vi "2_VisualizeModulePositioning2_Nolan.vi"(0 "Placement Monitor":T1(plugin-control)=refnum, 1 "Calibrated positions of fiducials [mm]":dbl[][](array[numeric])=[[-658.867386146, 115.937184375, -18.342965965], [-563.38738772, 115.95451918, -18.342965965], [-563.369748267, 18.796520782, -18.342965965], [-658.849746693, 18.779185977, -18.342965965], [-560.867387761, 115.954976697, -18.342965965], [-465.387389335, 115.972311502, -18.342965965], [-465.369749882, 18.814313103, -18.342965965], [-560.849748308, 18.796978298, -18.342965965], [-462.867389377, 115.972769019, -18.342965965], [-367.38739095, 115.990103824, -18.342965965], [-367.369751497, 18.832105425, -18.342965965], [-462.849749923, 18.81477062, -18.342965965], [-364.867390992, 115.990561341, -18.342965965], [-269.387392565, 116.007896146, -18.342965965], [-269.369753112, 18.849897747, -18.342965965], [-364.849751539, 18.832562942, -18.342965965], [-266.867392607, 116.008353663, -18.342965965], [-171.38739418, 116.025688468, -18.342965965], [-171.369754727, 18.867690069, -18.342965965], [-266.849753154, 18.850355264, -18.342965965], [-168.867394222, 116.026145985, -18.342965965], [-73.387395796, 116.04348079, -18.342965965], [-73.369756342, 18.885482391, -18.342965965], [-168.849754769, 18.868147586, -18.342965965], [-70.867395837, 116.043938306, -18.342965965], [24.612602589, 116.061273111, -18.342965965], [24.630242042, 18.903274713, -18.342965965], [-70.849756384, 18.885939908, -18.342965965], [27.132602548, 116.061730628, -18.342965965], [122.612600974, 116.079065433, -18.342965965], [122.630240427, 18.921067035, -18.342965965], [27.150242001, 18.90373223, -18.342965965], [125.132600933, 116.07952295, -18.342965965], [220.612599359, 116.096857755, -18.342965965], [220.630238812, 18.938859356, -18.342965965], [125.150240386, 18.921524551, -18.342965965], [223.132599318, 116.097315272, -18.342965965], [318.612597744, 116.114650077, -18.342965965], [318.630237197, 18.956651678, -18.342965965], [223.150238771, 18.939316873, -18.342965965], [321.132597702, 116.115107594, -18.342965965], [416.612596129, 116.132442399, -18.342965965], [416.630235582, 18.974444, -18.342965965], [321.150237156, 18.957109195, -18.342965965], [419.132596087, 116.132899916, -18.342965965], [514.612594514, 116.150234721, -18.342965965], [514.630233967, 18.992236322, -18.342965965], [419.15023554, 18.974901517, -18.342965965], [517.132594472, 116.150692238, -18.342965965], [612.612592899, 116.168027043, -18.342965965], [612.630232352, 19.010028644, -18.342965965], [517.150233925, 18.992693839, -18.342965965]], 2 "XYZ .NET Refnum in":refnum<k24>, 3 "Axis Speeds":T10={"X [mm/s]"=25.0, "Y [mm/s]"=25.0, "Z [mm/s]"=25.0}, 4 "Module fiducial marker":T7=enum."Mark C", 5 "N modules":i32=13, 6 "Sensor Pattern":T8(ring)=enum."ATLAS12", 7 "error in (no error)":errorcluster, 8 "Templates path":path=path "C:/Users/Aerotech/Documents/BNL_ThermomechanicalStave", 9 "Calibration [um/pix]":dbl=1.55, 10 "Current Build Phase":refnum<vi>, 11 "Temperature":refnum<vi>, 12 "Module #":refnum<vi>, 13 "Placement tolerance [um]":dbl=25.0, 14 "Tape Type":T5=enum."Axial (Sutcliffe NP49-01-100 01-Mar-16)", 16 "Module Report":refnum<vi>, 17 "Base notes":string, 18 "Reports path":path=path "C:/Users/Aerotech/cernbox/BNL/Stave Assembly Records/2017-05-15/ModulePlacement") -> (19 "Recalibrated??":bool, 22 "XYZ .NET Refnum out":refnum<k24>, 27 "error out":errorcluster)   [LabVIEW 2016]
uses:
  Utils/Controls/All_Enums/Enum_TypeDef_FidMarkers.ctl
  C:/Users/Aerotech/Documents/BNLStaveAssembly-blueprint/Bin/Aerotech.A3200.dll
  BNLStaveAssembly-blueprint/Bin/Aerotech.A3200.dll
  Utils/Controls/All_Enums/Enum_TypeDef_CornerSelection.ctl
  Utils/Controls/All_Enums/Enum_TypeDef_TapeType.ctl
panel:
  in  "Knob Turn Indicators":enum32{"Knob Turn Display", "Variables"}(tab)=enum."Variables"
  out "Corner A?":bool
  out "Corner B?":bool
  out "Corner C?":bool
  out "Corner D?":bool
  out "Y Knob Turns":dbl
  out "X Knob Turns":cluster{"X top ":dbl, "X bottom":dbl}
  out "Measured Coords":cluster{"X coordinate":sgl, "Y coordinate":sgl}
  out "Measured Coords 3":cluster{"X coordinate":sgl, "Y coordinate":sgl}
  out "Measured Coords 4":cluster{"X coordinate":sgl, "Y coordinate":sgl}
  out "Measured Coords 2":cluster{"X coordinate":sgl, "Y coordinate":sgl}
  out "True Coords":cluster{"X coordinate":dbl, "Y coordinate":dbl}
  out "True Coords 2":cluster{"X coordinate":dbl, "Y coordinate":dbl}
  out "True Coords 3":cluster{"X coordinate":dbl, "Y coordinate":dbl}
  out "True Coords 4":cluster{"X coordinate":dbl, "Y coordinate":dbl}
  out "Fiducial Template 2":T1(plugin-control)
  in  "Recalibrate!!":bool
  in  "Exit to survey or glue":bool
  out "Current task:":string="Applying glue for Module 11"
  in  "Tab Control: Positioning and Surveys":T2(tab)=enum."Apply glue"
  out "Offset interpreter":T3={"Offset Interpreter - Right"=FALSE, "Offset Interpreter - forward"=FALSE, "Offset Interpreter - backward"=TRUE, "Offset Interpreter - Left"=TRUE, "Placement Confirmation"=FALSE}
  in  "User Report: Current Module":T4={"B"=FALSE, "A"=FALSE, "D"=FALSE, "C"=FALSE, "ID"="", "Module #"=11, "x, centre"=368.8814166421462, "y, centre"=67.54477579693595, "Aligned"=FALSE, "Glue applied"=FALSE, "Placed"=FALSE}
  out "X offset [um]":sgl=497.0423
  out "Y offset [um]":sgl=417.2712
  in  "Module corner loop stop":bool
  in  "Center-only search?":bool
  in  "User notes":string="Type your note here...."
  out "Module # str":string="Module 11"
  in  "Assembly step":string(combo)
  in  "Manual Z?":bool
  in  "Manual Z [mm]":dbl
  in  "Dots (T) or Lines (F)":bool
  in  "Send XYZ stage beyond EOS":bool
  in  "Work on Corner...":T6=enum."[Exit]"
  in  "Work on Module #...":i32=11
  in  "Tab Control":enum32{"Fiducial marker", "Error reporting"}(tab)
  out "Fiducial Template":T1(plugin-control)
  out "Mark string":string="MarkC"
  out "Current Stage Position":T9={"X [mm]"=416.6304080435383, "Y [mm]"=18.974446486493466, "Z [mm]"=-18.342965704975803}
  out "Module Progress Report":T11(array[cluster])=[{"B"=FALSE, "A"=FALSE, "D"=FALSE, "C"=FALSE, "ID"="", "Module #"=1, "x, centre"=-611.1185672065, "y, centre"=67.3668525785, "Aligned"=FALSE, "Glue applied"=FALSE, "Placed"=FALSE}, {"B"=FALSE, "A"=FALSE, "D"=FALSE, "C"=FALSE, "ID"="", "Module #"=2, "x, centre"=-513.1185688215, "y, centre"=67.3846449, "Aligned"=FALSE, "Glue applied"=FALSE, "Placed"=FALSE}, {"B"=FALSE, "A"=FALSE, "D"=FALSE, "C"=FALSE, "ID"="", "Module #"=3, "x, centre"=-415.118570437, "y, centre"=67.402437222, "Aligned"=FALSE, "Glue applied"=FALSE, "Placed"=FALSE}, {"B"=FALSE, "A"=FALSE, "D"=FALSE, "C"=FALSE, "ID"="", "Module #"=4, "x, centre"=-317.118572052, "y, centre"=67.420229544, "Aligned"=FALSE, "Glue applied"=FALSE, "Placed"=FALSE}, {"B"=FALSE, "A"=FALSE, "D"=FALSE, "C"=FALSE, "ID"="", "Module #"=5, "x, centre"=-219.118573667, "y, centre"=67.438021866, "Aligned"=FALSE, "Glue applied"=FALSE, "Placed"=FALSE}, {"B"=FALSE, "A"=FALSE, "D"=FALSE, "C"=FALSE, "ID"="", "Module #"=6, "x, centre"=-121.118575282, "y, centre"=67.455814188, "Aligned"=FALSE, "Glue applied"=FALSE, "Placed"=FALSE}, {"B"=FALSE, "A"=FALSE, "D"=FALSE, "C"=FALSE, "ID"="", "Module #"=7, "x, centre"=-23.118576897500002, "y, centre"=67.4736065095, "Aligned"=FALSE, "Glue applied"=FALSE, "Placed"=FALSE}, {"B"=FALSE, "A"=FALSE, "D"=FALSE, "C"=FALSE, "ID"="", "Module #"=8, "x, centre"=74.8814214875, "y, centre"=67.4913988315, "Aligned"=FALSE, "Glue applied"=FALSE, "Placed"=FALSE}, {"B"=FALSE, "A"=FALSE, "D"=FALSE, "C"=FALSE, "ID"="", "Module #"=9, "x, centre"=172.8814198725, "y, centre"=67.509191153, "Aligned"=FALSE, "Glue applied"=FALSE, "Placed"=FALSE}, {"B"=FALSE, "A"=FALSE, "D"=FALSE, "C"=FALSE, "ID"="", "Module #"=10, "x, centre"=270.8814182575, "y, centre"=67.52698347500001, "Aligned"=FALSE, "Glue applied"=FALSE, "Placed"=FALSE}, {"B"=FALSE, "A"=FALSE, "D"=FALSE, "C"=FALSE, "ID"="", "Module #"=11, "x, centre"=368.8814166421462, "y, centre"=67.54477579693595, "Aligned"=FALSE, "Glue applied"=FALSE, "Placed"=FALSE}, {"B"=FALSE, "A"=FALSE, "D"=FALSE, "C"=FALSE, "ID"="", "Module #"=12, "x, centre"=466.881415027, "y, centre"=67.562568119, "Aligned"=FALSE, "Glue applied"=FALSE, "Placed"=FALSE}, {"B"=FALSE, "A"=FALSE, "D"=FALSE, "C"=FALSE, "ID"="", "Module #"=13, "x, centre"=564.881413412, "y, centre"=67.580360441, "Aligned"=FALSE, "Glue applied"=FALSE, "Placed"=FALSE}]
  # "VISUALIZE MODULE PLACEMENT Brandeis University - Brookhaven National Laboratory * ATLAS Phase II Inner Tracker Upgrade * Primary Authors: Hannah Herde (hherde@brandeis.edu), Laura Bergsten (lbergsten@brandeis.edu)"
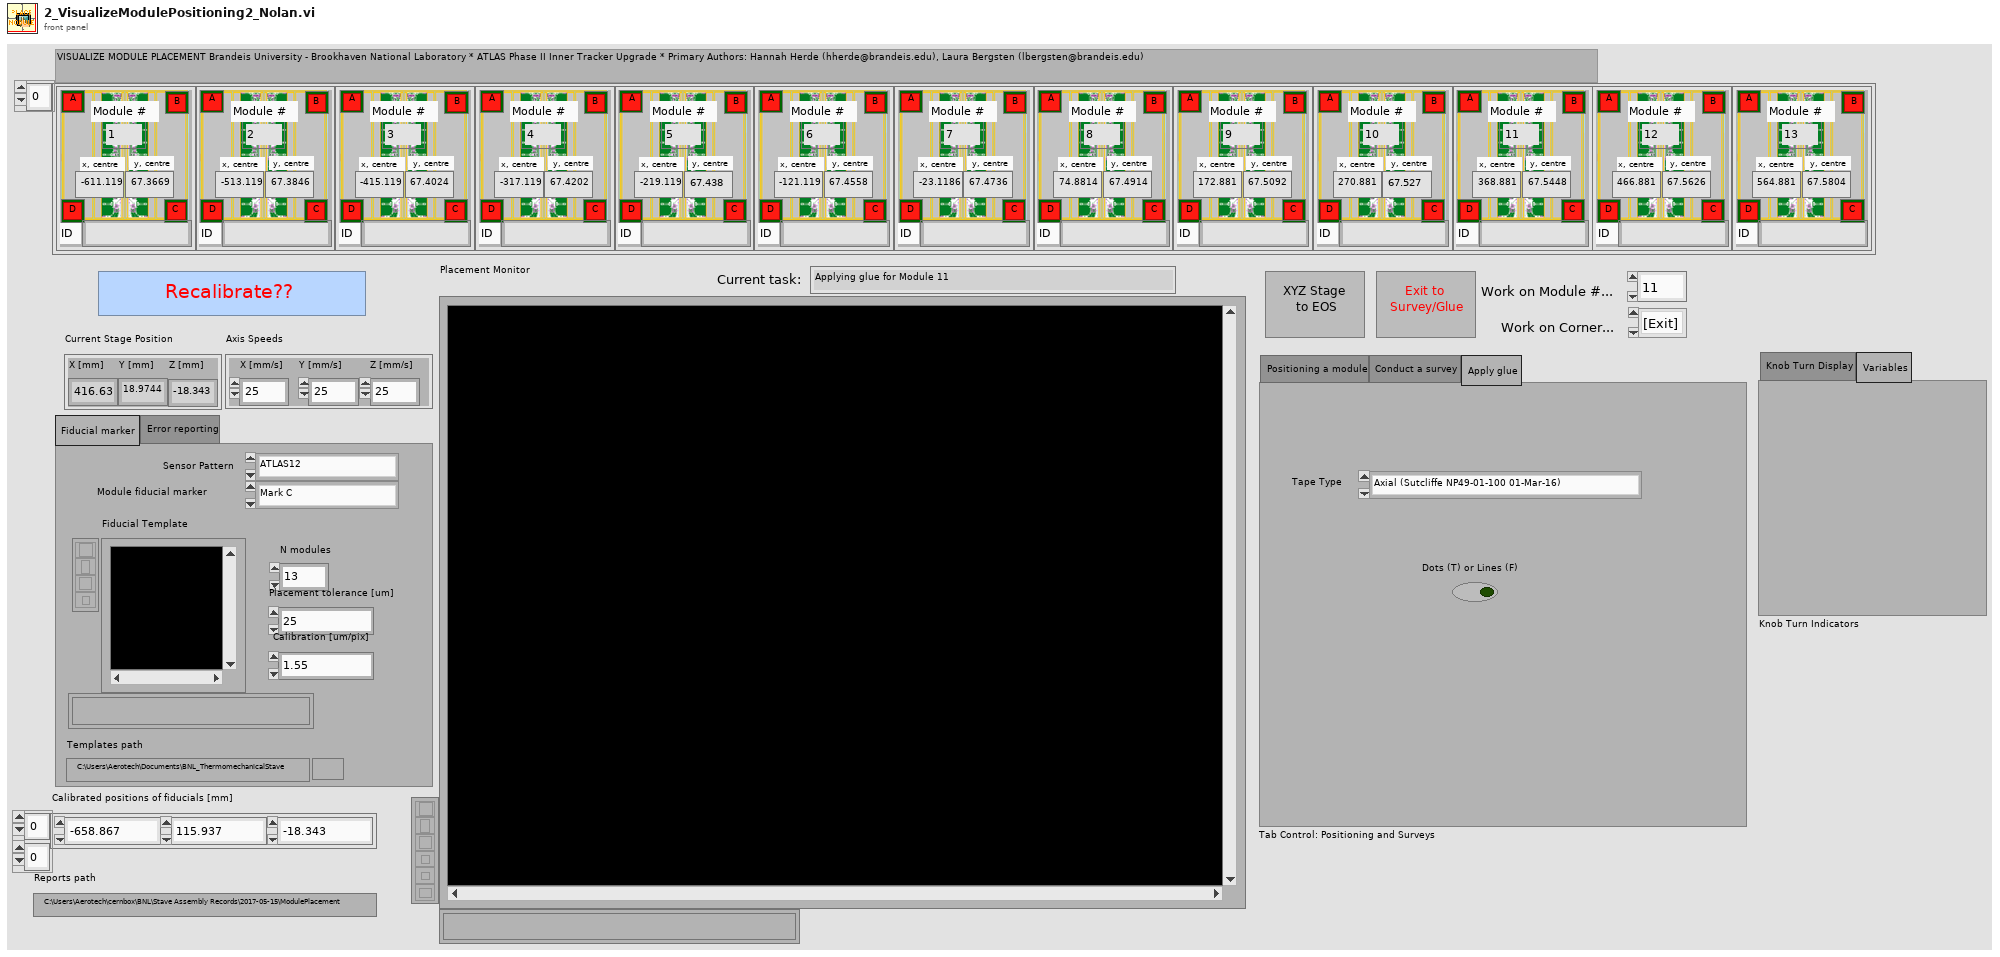
[diagram p1: front panel]
types:
  T1 = typedef "IMAQ Image.ctl" = refnum<image>
  T2 = enum32{"Positioning a module", "Conduct a survey", "Apply glue"}
  T3 = cluster{"Offset Interpreter - Right":bool, "Offset Interpreter - forward":bool, "Offset Interpreter - backward":bool, "Offset Interpreter - Left":bool, "Placement Confirmation":bool}
  T4 = cluster{"B":bool, "A":bool, "D":bool, "C":bool, "ID":string, "Module #":i32, "x, centre":dbl, "y, centre":dbl, "Aligned":bool, "Glue applied":bool, "Placed":bool}
  T5 = typedef "Enum_TypeDef_TapeType.ctl" = enum16{"Right stereo", "Left stereo", "Stereo (Sutcliffe NP49-01-100 01-Mar-16)", "Axial (Sutcliffe NP49-01-100 01-Mar-16)"}
  T6 = typedef "Enum_TypeDef_CornerSelection.ctl" = enum16{"A", "B", "C", "D", "[Exit]"}
  T7 = typedef "Enum_TypeDef_FidMarkers.ctl" = enum16{"Mark B", "Mark C", "Bias Ring Corner", "Mark I (Slim/17)", "Mark E (Slim/17)", "Mark F (Slim/17)", "Mark G (Slim/17)", "Mark A (12)", "Kapton Spacers"}
  T8 = enum16{"ATLAS07", "ATLAS12", "ATLAS12Slim", "ATLAS17LS"}
  T9 = cluster{"X [mm]":dbl, "Y [mm]":dbl, "Z [mm]":dbl}
  T10 = cluster{"X [mm/s]":dbl, "Y [mm/s]":dbl, "Z [mm/s]":dbl}
  T11 = cluster{"B":bool, "A":bool, "D":bool, "C":bool, "ID":string, "Module #":i32, "x, centre":dbl, "y, centre":dbl, "Aligned":bool, "Glue applied":bool, "Placed":bool}[]
  T12 = enum8{"Enabled", "Disabled", "Disabled and Grayed Out"}
  T13 = enum16{"Left Button", "Center Button", "Right Button", "Window Close"}
  T14 = cluster{"Final X":dbl, "Final Y":dbl, "Final Z":dbl}
  T15 = cluster{"Measured Coords":cluster{"X coordinate":sgl, "Y coordinate":sgl}, "Measured Coords 2":cluster{"X coordinate":sgl, "Y coordinate":sgl}, "Measured Coords 3":cluster{"X coordinate":sgl, "Y coordinate":sgl}, "Measured Coords 4":cluster{"X coordinate":sgl, "Y coordinate":sgl}}
  T16 = cluster{"True Coords":cluster{"X coordinate":dbl, "Y coordinate":dbl}, "True Coords 2":cluster{"X coordinate":dbl, "Y coordinate":dbl}, "True Coords 3":cluster{"X coordinate":dbl, "Y coordinate":dbl}, "True Coords 4":cluster{"X coordinate":dbl, "Y coordinate":dbl}}
  T17 = cluster{"ID":string, "Mark string":string, "Assembly step":string, "User notes":string, string, "Corner surveyed position":dbl[]}
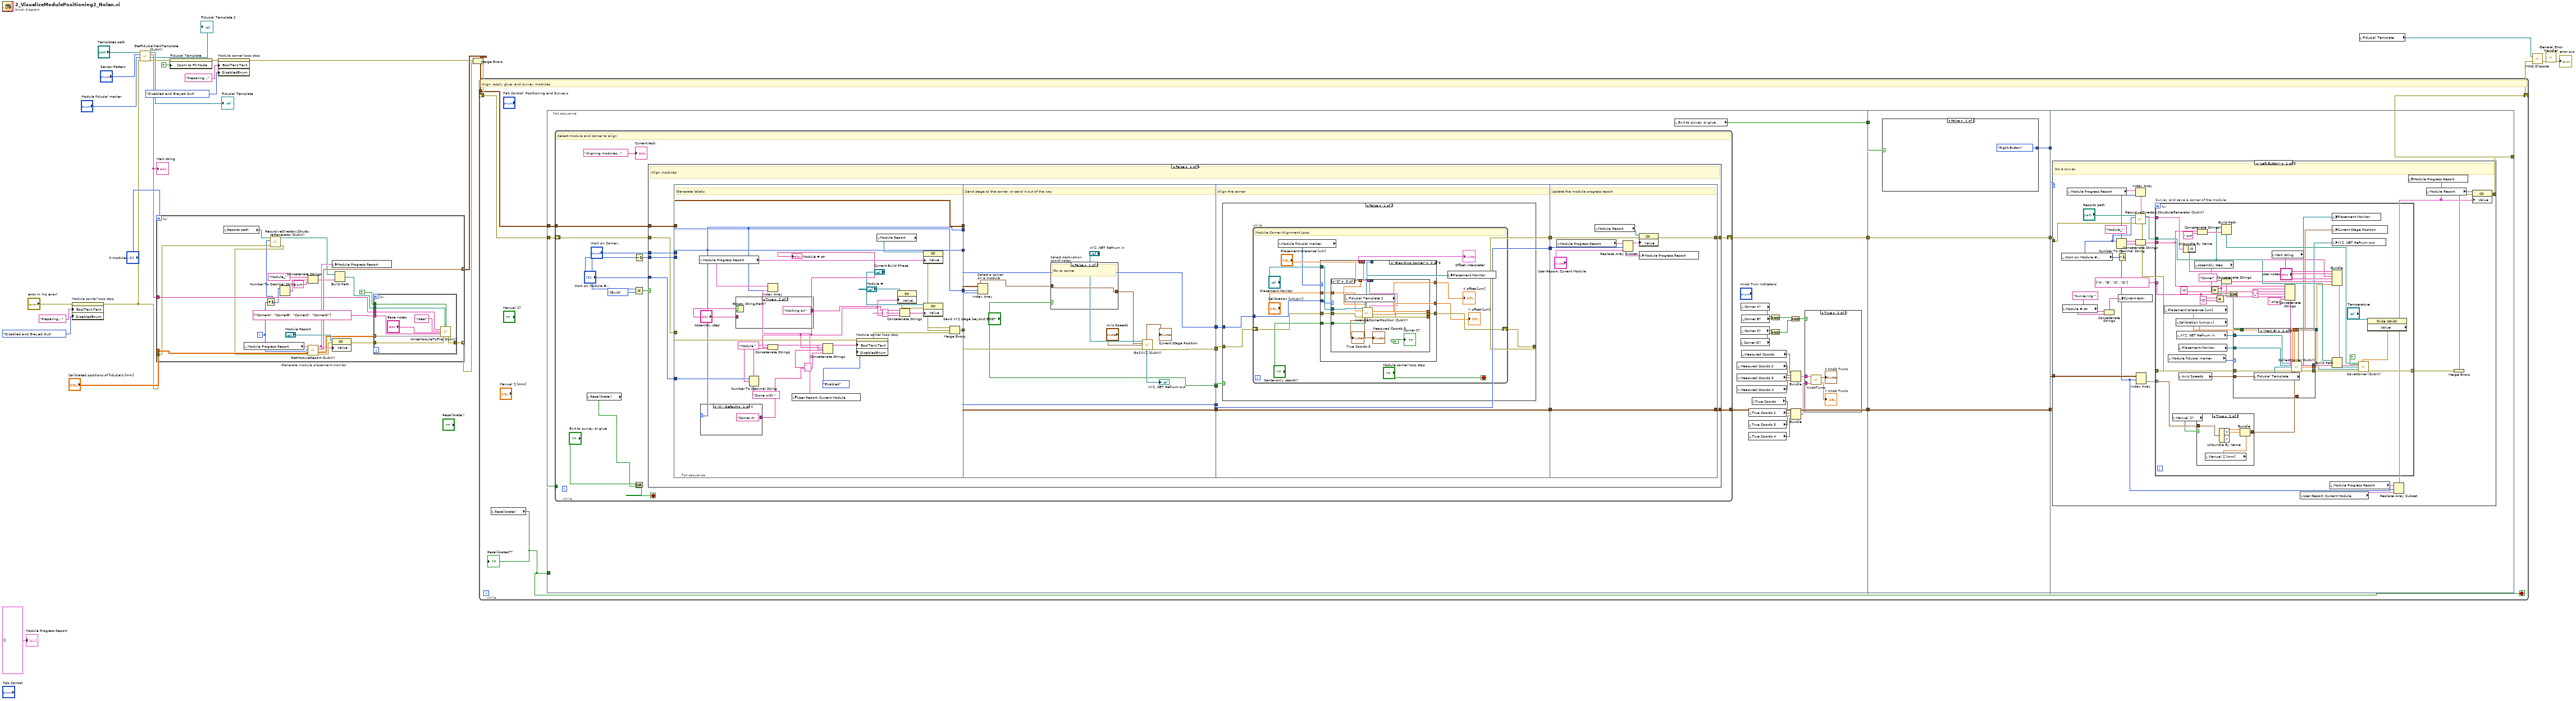
[diagram p0: block diagram]
diagram:
  n1 = property on="Module corner loop stop" class="Bool"(error in="error in (no error)", "BoolText.Text"="Preparing..." ("Boolean Text.Text"), "DisabledEnum"=T12."Disabled and Grayed Out" ("Disabled")) -> (error out=w13:errorcluster)  [unwired: 1 in, 1 out]
  n2 = call "GetFiducialMarkTemplate (SubVI).vi"("error in (no error)"=w13, "Module fiducial marker"="Module fiducial marker", "Sensor Pattern"="Sensor Pattern", "Templates path"="Templates path") -> ("error out"=w17:errorcluster, "Template out 2"=→"Fiducial Template 2":T1, "Mark string"=w3:string, "Template out"=→"Fiducial Template":T1)  [unwired: 4 in]
  "Mark string" <- w3
  n3 = for "Generate module placement monitor" {
    N: "N modules" -> [_]
    tunnel: "Calibrated positions of fiducials [mm]" -> [w49]
    tunnel: [w48] -> w10 mode=indexing
    tunnel: w13 -> [w29]
    tunnel: [w37] -> w2 mode=indexing
    tunnel: w3 -> [w33]
    i -> [w32]
    n4 = local read "Reports path"() -> (w31:path)
    n5 = local read "Module Progress Report"() -> (w44:T11)
    n6 = Increment(x=w32) -> (x+1=w27:i32)
    n7 = call "RecursiveDirectoryStructureGenerator (SubVI).vi"("error in (no error)"=w29, "Folder index"=w27, "Host directory"=w31) -> ("error out"=w28:errorcluster, "Nth subfolder in host directory"=w30:path)  [unwired: 7 in]
    n8 = Number To Decimal String(number=w27) -> (decimal integer string=w42:string)  [unwired: 1 in]
    n9 = Concatenate Strings("Module_" ("string"), w42, ".txt" ("string")) -> (w40:string)
    n10 = call "GetModuleReport (SubVI).vi"("error in (no error)"=w28, "Calibrated positions of fiducials [mm]"=w49, "ith Module"=w32, "Module Progress Report in"=w44) -> ("error out"=w46:errorcluster, "MyCorners"=w38:dbl[][], "Array of ith module cluster fiducial mark positions"=w48:cluster{"X":dbl, "Y":dbl, "Z":dbl}[], "Module Progress Report out"=w47:T11)  [unwired: 4 in]
    n11 = local write "Module Progress Report"(w47) -> ()
    n12 = property class="Ctl"(reference="Module Report", error in=w46, "Value"=w47) -> (error out=w36:errorcluster)  [unwired: 1 out]
    n13 = Build Path(base path=w30, name or relative path=w40) -> (appended path=w34:path)
    n14 = for {
      tunnel: string[] ["CornerA", "CornerB", "CornerC", "CornerD"] -> [w58] mode=indexing
      tunnel: w38 -> [w57] mode=indexing
      tunnel: [w56] -> w37
      tunnel: w36 -> [w55]
      tunnel: TRUE ("Write to file") -> [w54]
      tunnel: w34 -> [w53]
      tunnel: w33 -> [w52]
      n15 = call "WriteModuleToFile (SubVI).vi"("Mark used for tracking"=w52, "Assembly step"="Ideal", "User notes"="Base notes", "Current corner"=w58, "Fiducial Mark Position"=w57, "error in (no error)"=w55, "Module reports file path"=w53, "Write to file"=w54) -> ("error out"=w56:errorcluster)  [unwired: 11 in]
    }
  }
  n16 = property on="Fiducial Template" class="ImageControl"(error in=w17, "Zoom to Fit Mode"=TRUE) -> (error out=w9:errorcluster)  [unwired: 1 in, 1 out]
  n17 = property on="Module corner loop stop" class="Bool"(error in=w9, "BoolText.Text"="Preparing..." ("Boolean Text.Text"), "DisabledEnum"=T12."Disabled and Grayed Out" ("Disabled")) -> (error out=w4:errorcluster)  [unwired: 1 in, 1 out]
  n18 = Merge Errors(w4, w2) -> (w6:errorcluster)
  n19 = while {
    tunnel: w10 -> [w67]
    shift-right: [w63] -> w5
    shift-left: w6 -> [w66]
    stop <- w59 stop-if-true
    # "Align, apply glue, and survey modules"
    n20 = local read "Recalibrate!!"() -> (w59:bool)
    "Recalibrated??" <- w59
    n21 = flat-sequence {
      tunnel: w67 -> [w91]
      tunnel: w66 -> [w89]
      tunnel: [w90] -> w64
      tunnel: [w88] -> w62
      tunnel: w59 -> [w87]
      tunnel: [w86] -> w60
      tunnel: [w406] -> w68
      tunnel: [w405] -> w65
      tunnel: w64 -> [w405]
      tunnel: w62 -> [w404]
      tunnel: [w404] -> w61
      tunnel: w60 -> [w403]
      tunnel: w68 -> [w422]
      tunnel: w65 -> [w421]
      tunnel: [w420] -> w63
      tunnel: w61 -> [w419]
      frame #0 {
        n22 = while {
          tunnel: w91 -> [w103]
          tunnel: [w102] -> w90
          shift-right: [w100] -> w88
          shift-left: w89 -> [w99]
          tunnel: w87 -> [_]
          stop <- w97 stop-if-true
          # "Select module and corner to align"
          n23 = local read "Recalibrate!!"() -> (w96:bool)
          n24 = Equal?(x="Work on Corner...", y=enum16{"A", "B", "C", "D", "[Exit]"}."[Exit]") -> (x = y?=w106:bool)
          n25 = Or(x="Exit to survey or glue", y=w96) -> (x .or. y?=w97:bool)
          n26 = Decrement(x="Work on Module #...") -> (x-1=w104:i32)
          n27 = case shown="False" w106 {
            tunnel: "Work on Corner..." -> [w128 _]
            tunnel: w104 -> [w126 w379]
            tunnel: w103 -> [w124 w380]
            tunnel: [w118 w380] -> w102
            tunnel: "Work on Module #..." -> [w117 _]
            tunnel: w99 -> [w116 w378]
            tunnel: [w112 w376] -> w100
            frame False {
              # "Align modules"
              n28 = flat-sequence {
                tunnel: w128 -> [w129]
                tunnel: [w129] -> w127
                tunnel: w126 -> [w136]
                tunnel: [w137] -> w125
                tunnel: w124 -> [w137]
                tunnel: [w136] -> w123
                tunnel: w117 -> [w135]
                tunnel: w116 -> [w134]
                tunnel: [w133] -> w115
                tunnel: [w129] -> w109
                tunnel: w127 -> [w170]
                tunnel: w125 -> [w168]
                tunnel: w123 -> [w169]
                tunnel: [w169] -> w121
                tunnel: [w168] -> w119
                tunnel: w115 -> [w167]
                tunnel: [w166] -> w114
                tunnel: ["Send XYZ stage beyond EOS"] -> w111
                tunnel: [w164] -> w110
                tunnel: w109 -> [w164]
                tunnel: [w183] -> w122
                tunnel: w121 -> [w183]
                tunnel: [w182] -> w120
                tunnel: w119 -> [w182]
                tunnel: w114 -> [w181]
                tunnel: [w180] -> w113
                tunnel: w111 -> [w179]
                tunnel: w110 -> [w178]
                tunnel: w122 -> [w370]
                tunnel: w120 -> [w369]
                tunnel: [w369] -> w118
                tunnel: w113 -> [w368]
                tunnel: [w367] -> w112
                frame #0 {
                  # "Generate labels"
                  n29 = local read "Module Progress Report"() -> (w139:T11)
                  n30 = case shown="\"A\", Default" w129 {
                    tunnel: ["Corner A" "Corner B" "Corner C" "Corner D"] -> w152
                    frame "A", Default {
                    }
                    frame "B" {
                    }
                    frame "C" {
                    }
                    frame "D" {
                    }
                  }
                  n31 = Empty String/Path?(string/path="Assembly step") -> (empty?=w132:bool)
                  n32 = case shown="True" w132 {
                    tunnel: [w157 "Working on" ("Assembly step")] -> w130
                    tunnel: "Assembly step" -> [w157 _]
                    frame False {
                    }
                    frame True {
                    }
                  }
                  n33 = Number To Decimal String(number=w135) -> (decimal integer string=w147:string)  [unwired: 1 in]
                  n34 = Index Array(array=w139, index=w136) -> (element=w138:T4)
                  n35 = Concatenate Strings("Module " ("string"), w147) -> (w153:string)
                  "Module # str" <- w153
                  n36 = local write "User Report: Current Module"(w138) -> ()
                  n37 = Concatenate Strings("Done with " ("string"), w153, ",  " ("string"), w152) -> (w151:string)
                  n38 = property on="Module corner loop stop" class="Bool"(error in=w134, "BoolText.Text"=w151, "DisabledEnum"=T12."Enabled" ("Disabled")) -> (error out=w156:errorcluster)  [unwired: 1 in, 1 out]
                  n39 = local read "Module Report"() -> (w140:refnum<vi>)
                  n40 = property class="Str"(reference="Module #", "Value"=w153) -> (error out=w144:errorcluster)  [unwired: 1 in, 1 out]
                  n41 = Concatenate Strings(w130, ": " ("string"), w153) -> (w145:string)
                  n42 = property class="Ctl"(reference=w140, "Value"=w139) -> (error out=w155:errorcluster)  [unwired: 1 in, 1 out]
                  n43 = property class="Str"(reference="Current Build Phase", error in=w144, "Value"=w145) -> (error out=w154:errorcluster)  [unwired: 1 out]
                  n44 = Merge Errors(w155, w154, w156) -> (w133:errorcluster)
                }
                frame #1 {
                  # "Send stage to the corner, or send it out of the way"
                  n45 = Index Array "Select a corner\non a module"(array=w168, index (row)=w169, index (col)=w170) -> (element=w163:cluster{"X":dbl, "Y":dbl, "Z":dbl})
                  n46 = case "Select destination coordinates" shown="False" "Send XYZ stage beyond EOS" {
                    tunnel: [w176 cluster{"X":dbl, "Y":dbl, "Z":dbl} {"X"=-725.0, "Y"=0.0, "Z"=-49.0}] -> w172
                    tunnel: w163 -> [w176 _]
                    frame False {
                      # "Go to corner"
                    }
                    frame True {
                      # "Send stage away"
                    }
                  }
                  n47 = call "Go2XYZ (SubVI).vi"(".NET Refnum in"="XYZ .NET Refnum in", "Go to Coordinates"=w172, "Axis Speeds"="Axis Speeds", "error in (no error)"=w167) -> (".NET Refnum out"=→"XYZ .NET Refnum out":refnum<k24>, "Final Position"=→"Current Stage Position":T14, "error out"=w166:errorcluster)  [unwired: 7 in, 2 out]
                }
                frame #2 {
                  # "Align the corner"
                  n48 = case shown="False" w179 {
                    tunnel: w181 -> [w186 w366]
                    tunnel: [w185 w366] -> w180
                    tunnel: w178 -> [w184 _]
                    frame False {
                      n49 = while "Module Corner Placement Loop" {
                        shift-right: [w198] -> w185
                        shift-left: w186 -> [w190]
                        tunnel: w184 -> [w188]
                        stop <- "Module corner loop stop" stop-if-true
                        # "Module Corner Alignment Loop"
                        n50 = local read "Module fiducial marker"() -> (w187:T7)
                        n51 = case shown="\"Bias Ring Corner\"" w187 {
                          tunnel: [w208 w220 w297 w308 w319 w330 w341 w352 w365] -> w198
                          tunnel: [w204 w216 w293 w304 w315 w326 w337 w348 w364] -> w197
                          tunnel: "Placement tolerance [um]" -> [w203 w215 w292 w303 w314 w325 w336 w347 w363]
                          tunnel: "Placement Monitor" -> [w205 w217 w294 w305 w316 w327 w338 w349 w362]
                          tunnel: "Calibration [um/pix]" -> [w201 w213 w290 w301 w312 w323 w334 w345 w361]
                          tunnel: [w202 w214 w291 w302 w313 w324 w335 w346 w360] -> w193
                          tunnel: [w206 w218 w295 w306 w317 w328 w339 w350 w359] -> w192
                          tunnel: [w207 w219 w296 w307 w318 w329 w340 w351 w358] -> w191
                          tunnel: w190 -> [w209 w221 w298 w309 w320 w331 w342 w353 w357]
                          tunnel: "Center-only search?" -> [w200 w212 w289 w300 w311 w322 w333 w344 w356]
                          tunnel: w188 -> [_ w211 _ _ _ _ _ _ _]
                          frame "Mark B", Default {
                            n52 = local read "Fiducial Template"() -> (w210:T1)
                            n53 = call "AnalyzeCornerPosition (SubVI).vi"("Refnum in"=w205, "Placement tolerance [um]"=w203, "Calibration [um/pix]"=w201, "Fiducial Template"=w210, "error in (no error)"=w209, "Center-only search?"=w200) -> ("Offset interpreter"=w202:T3, "Refnum out"=w204:T1, "X offset [um]"=w206:sgl, "Y offset [um]"=w207:sgl, "error out"=w208:errorcluster)  [unwired: 3 in, 2 out]
                          }
                          frame "Bias Ring Corner" {
                            n54 = case shown="\"C\"" w211 {
                              tunnel: w221 -> [w234 w248 w262 w276 w287]
                              tunnel: [w233 w247 w261 w275 w286] -> w220
                              tunnel: [w232 w246 w260 w274 w285] -> w219
                              tunnel: [w231 w245 w259 w273 w284] -> w218
                              tunnel: w217 -> [w230 w244 w258 w272 w283]
                              tunnel: [w229 w243 w257 w271 w282] -> w216
                              tunnel: w215 -> [w228 w242 w256 w270 w281]
                              tunnel: [w227 w241 w255 w269 w280] -> w214
                              tunnel: w213 -> [w226 w240 w254 w268 w279]
                              tunnel: w212 -> [w225 w239 w253 w267 w278]
                              frame "B" {
                                n55 = local read "Fiducial Template"() -> (w235:T1)
                                n56 = call "AnalyzeCornerPosition (SubVI).vi"("Refnum in"=w230, "Placement tolerance [um]"=w228, "Calibration [um/pix]"=w226, "Fiducial Template"=w235, "error in (no error)"=w234, "Center-only search?"=w225) -> ("Offset interpreter"=w227:T3, "Refnum out"=w229:T1, "X offset [um]"=w231:sgl, "Y offset [um]"=w232:sgl, "True Coords"=→"True Coords 2":cluster{"X coordinate":dbl, "Y coordinate":dbl}, "Measured Coords"=→"Measured Coords 2":cluster{"x":sgl, "y":sgl}, "error out"=w233:errorcluster)  [unwired: 3 in]